vi "Main.vi"() -> ()   [LabVIEW 2020]
uses:
  Global_Variable/Global.vi
  Database/Global1.vi
  Global_Variable/A131258.vi
  <userlib>/_MGI/Menu Building/MenuTypes/MenuStrip/MGI_MenuStrip.lvclass
  <userlib>/_MGI/Menu Building/MenuItemStatusChange/MGI_MenuItemStatusChange.lvclass
  System.Windows.Forms
panel:
  in  "表格控件":string[][](table)
  out "上序状态":string
  in  "Andon":enum32{"未选择", "缺料报警", "质量报警", "故障报警"}(radio)
  in  "菜单":refnum<k24>(container)
  out "试验计时":u16
  out "工位传感器码":string
  out "生产数量":i32
  out "合格数量":i32
  out "userStatus":string caption="用户状态"
  out "userName":string caption="用户名"
  out "connectionMode":string caption="联机类型"
  out "产品型号":string
  in  "更换产品":refnum<vi>
  out "提示信息":string
  out "错误":bool
  out "时间字符串":string
  out "日期字符串":string
  out "自动":bool
  # "上转向轴组件压装"
  # "实验项目"
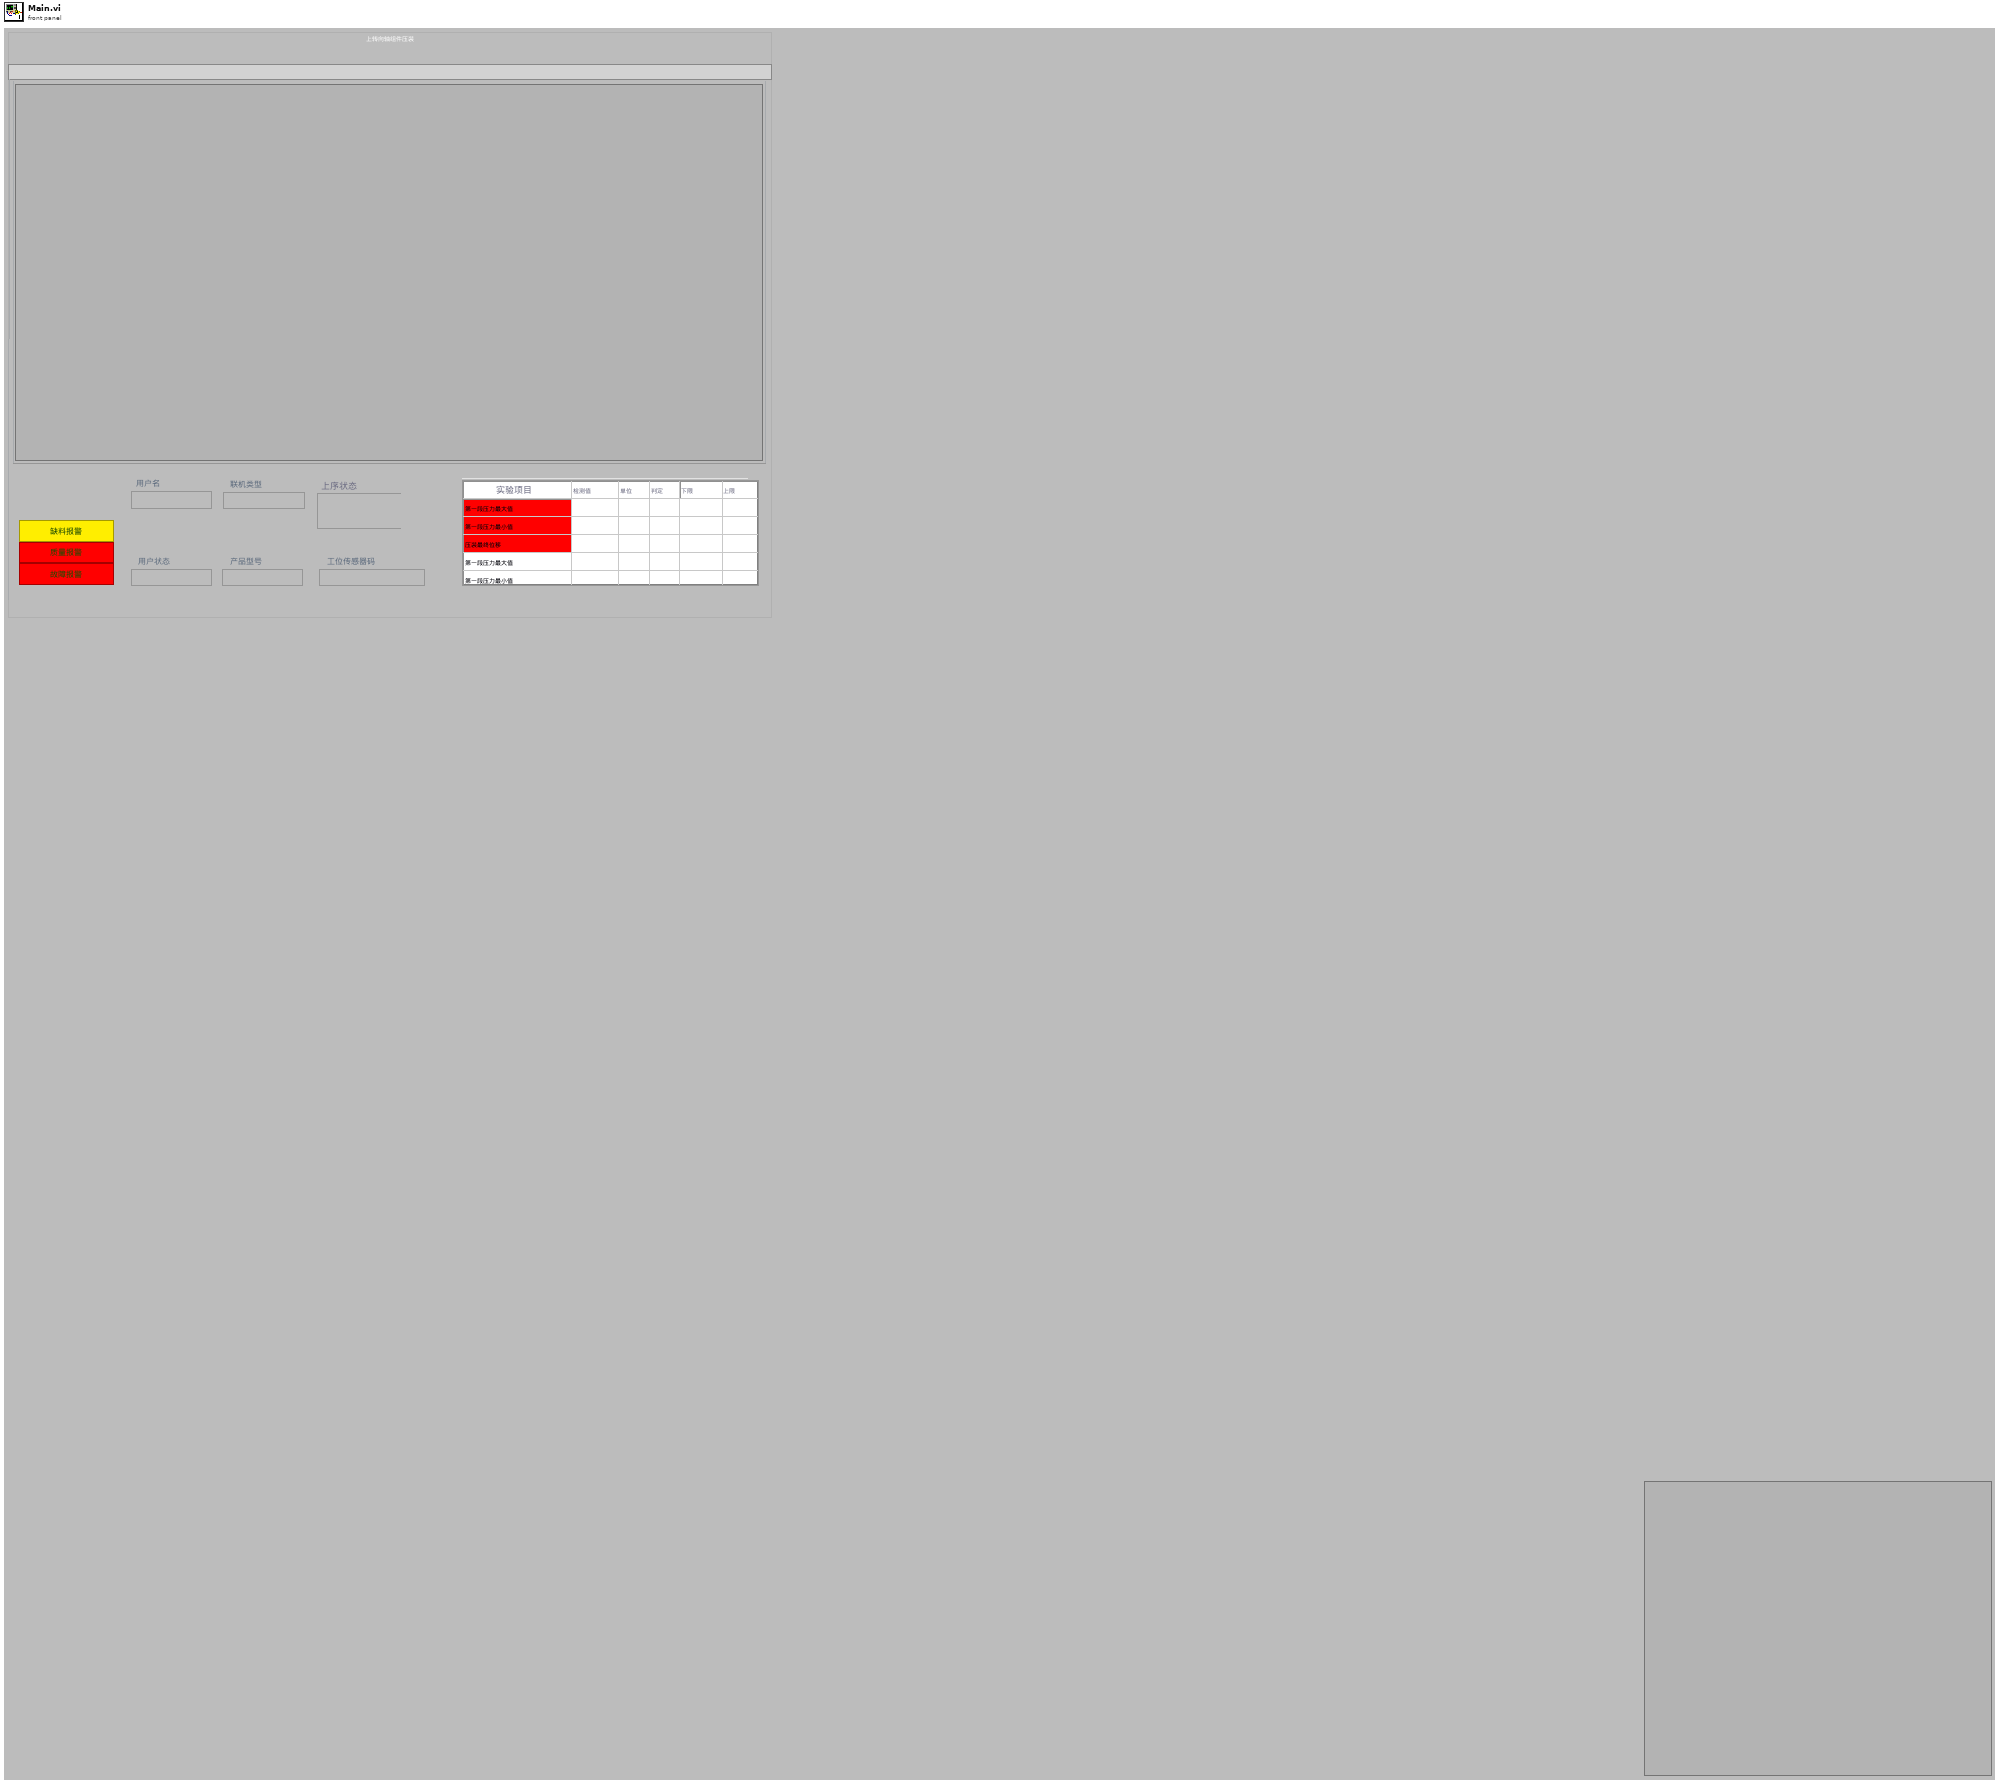
[diagram p1: front panel]
types:
  T1 = enum32{"Invalid", "Standard", "Closed", "Hidden", "Minimized", "Maximized"}
  T2 = cluster{"设备名称":string, "操作人员":string, "设备状态":enum16{"设备离线", "设备正常", "设备缺料", "设备故障", "质量报警"}, "附加信息":string}
  T3 = enum32{"invalid app kind", "Development System", "Run Time System", "Student Edition", "Embedded LabVIEW", "Evaluation", "Custom"}
  T4 = cluster{"用户编号":string, "用户名":string, "用户密码(密文)":string, "用户权限":string}
  T5 = cluster{"Core":cluster{"Current VI Reference":refnum<vi>, "Close Panel on Exit?":bool}, "Your Boolean data":bool, "Your string data":string}
  T6 = cluster{"Current VI Reference":refnum<vi>, "Close Panel on Exit?":bool}
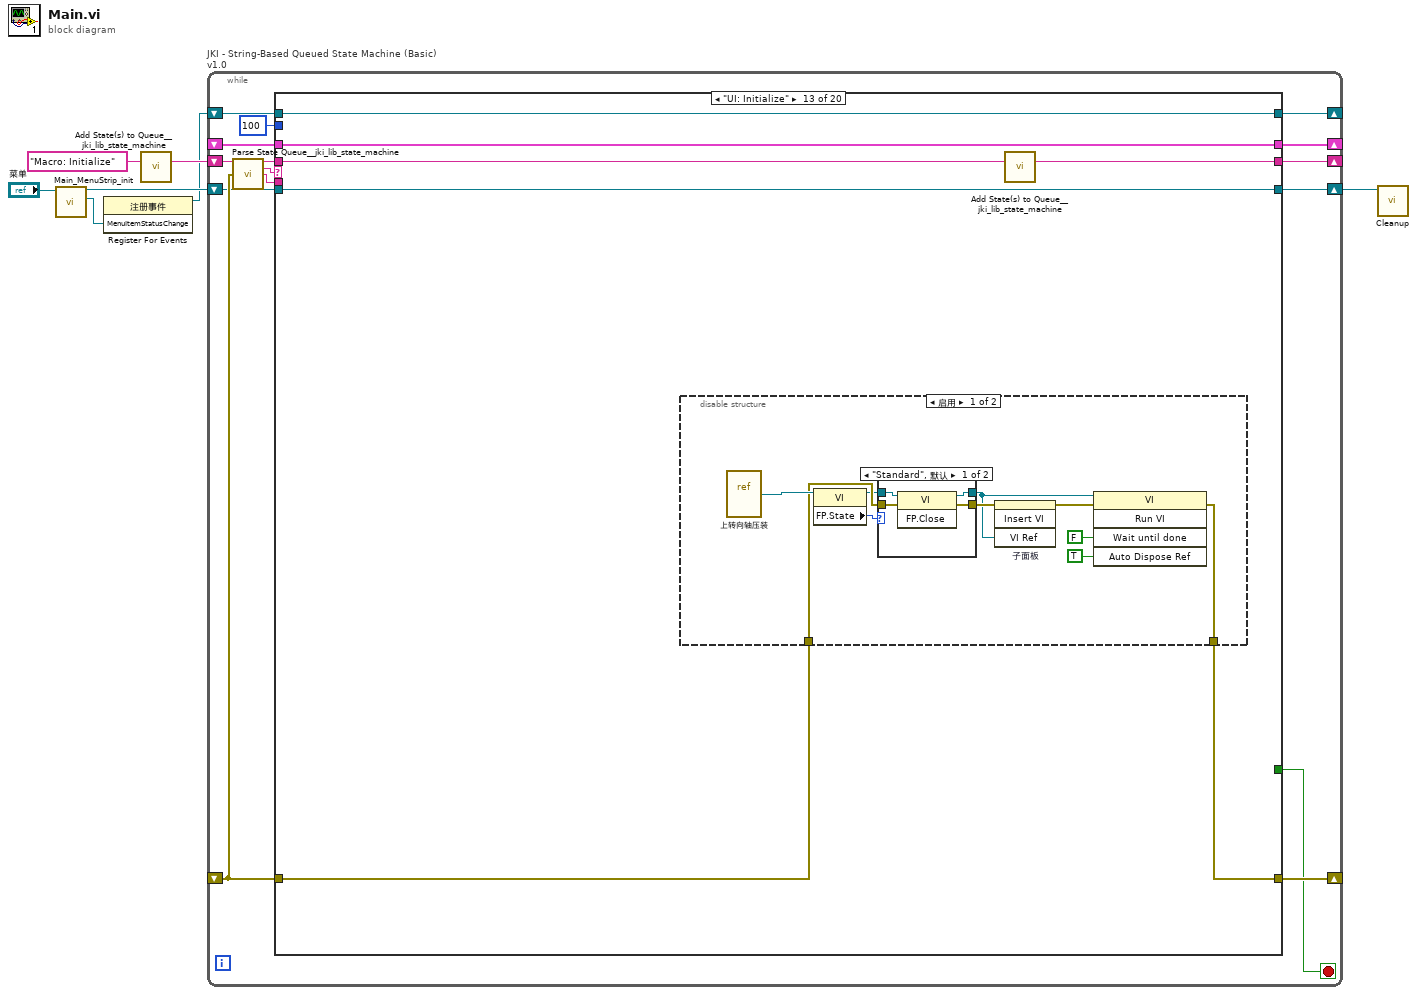
[diagram p0: block diagram]
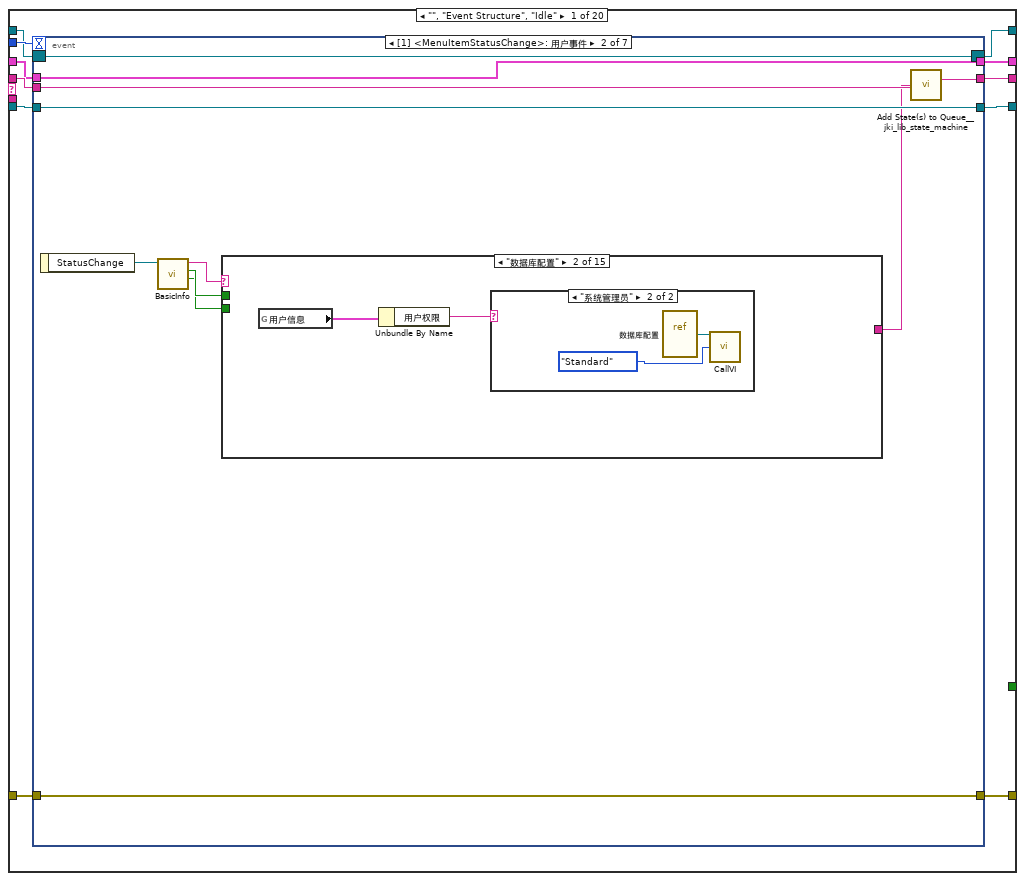
[diagram p2: hidden frame]
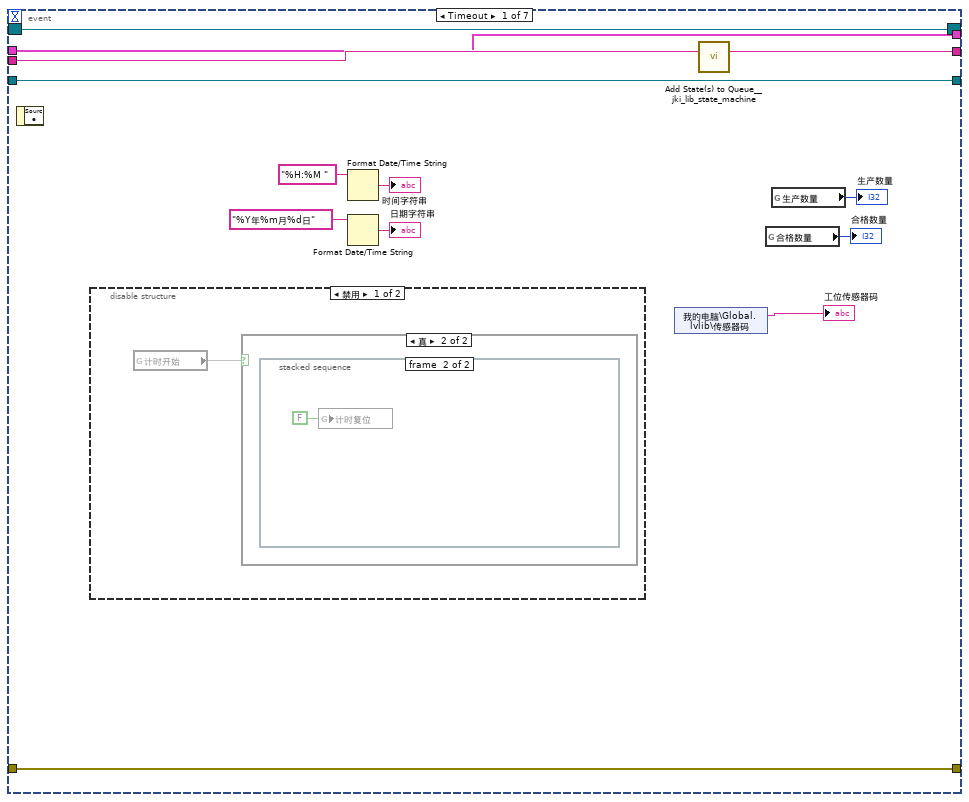
[diagram p3: hidden frame]
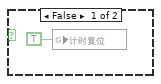
[diagram p4: hidden frame]
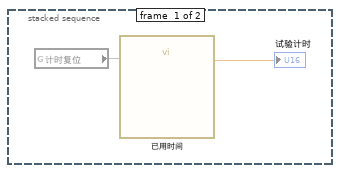
[diagram p5: hidden frame]
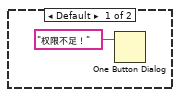
[diagram p8: hidden frame]
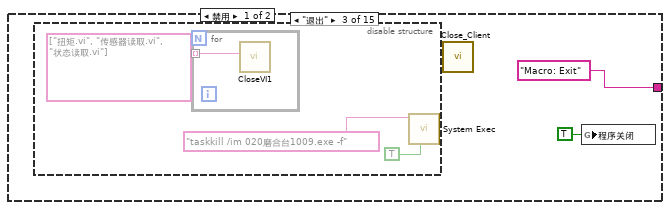
[diagram p9: hidden frame]
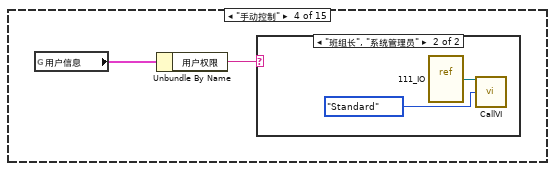
[diagram p11: hidden frame]
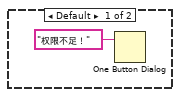
[diagram p12: hidden frame]
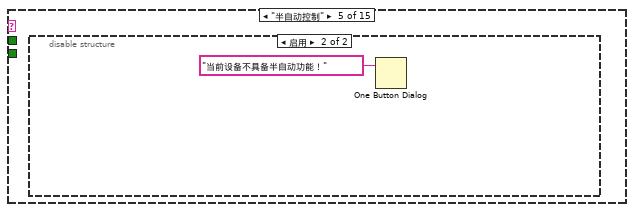
[diagram p13: hidden frame]
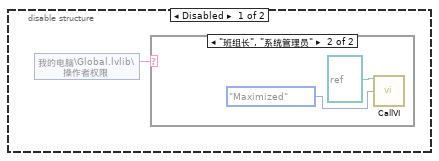
[diagram p14: hidden frame]
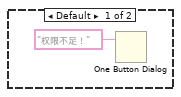
[diagram p15: hidden frame]
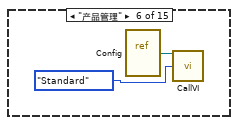
[diagram p16: hidden frame]
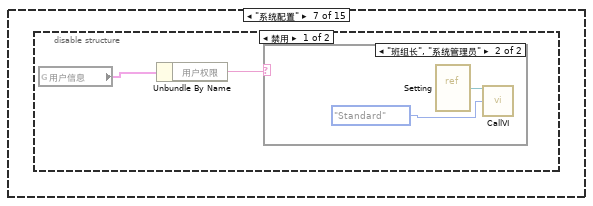
[diagram p17: hidden frame]
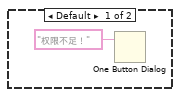
[diagram p18: hidden frame]
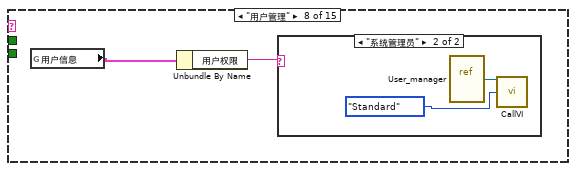
[diagram p20: hidden frame]
diagram:
  n1 = call "Main_MenuStrip_init.vi"("MenuStrip"="菜单") -> ("MenuItemStatusChange"=w2:refnum<user-event>, "Menu out"=w4:refnum<class "MGI_MenuStrip.lvclass">)  [unwired: 9 in]
  n2 = register-events(w2) -> (reference out=w1:refnum<event-registration>)  [unwired: 2 in, 1 out]
  n3 = call <vilib>:"Add State(s) to Queue__jki_lib_state_machine.vi"("State(s) in (\"\")"="Macro: Initialize") -> ("States Out"=w7:string)  [unwired: 14 in]
  n4 = while "JKI - String-Based Queued State Machine (Basic) v1.0" {
    shift-right: [w16] -> _
    shift-left: _ -> [w15]
    shift-right: [w18] -> _
    shift-left: _ -> [w13]
    shift-right: [w17] -> _
    shift-left: w7 -> [w19]
    shift-right: [w11] -> w3
    shift-left: w4 -> [w12]
    shift-right: [w9] -> _
    shift-left: w1 -> [w8]
    stop <- w10 stop-if-true
    n5 = call <vilib>:"Parse State Queue__jki_lib_state_machine.vi"("State Queue"=w19, "Error In (no error)"=w13) -> ("Remaining States"=w21:string, "Current State"=w22:string, "Arguments"=w20:string)  [unwired: 11 in]
    n6 = case shown="\"UI: Initialize\"" w22 {
      selector: w22 -> [_ _ w190 _ _ _ _ _ _ _ _ _ _ _ _ _ _ _ _ _]
      tunnel: w21 -> [w33 w187 w194 w214 w222 w229 w235 w238 w246 w257 w265 w271 w278 w302 w343 w351 w364 w392 w399 w411]
      tunnel: w20 -> [_ _ _ _ _ _ _ _ _ _ _ _ _ _ _ w346 w358 _ _ _]
      tunnel: w15 -> [w31 w184 w192 w205 w219 w227 w232 w239 w243 _ w260 w268 w276 w300 w340 w349 w360 w389 w396 w408]
      tunnel: [w30 w185 w196 w211 errorcluster {"status"=FALSE, "code"=0, "source"=""} ("error out") w226 w233 w236 w244 w254 w261 w269 w275 w298 w341 w347 w361 w390 w397 w409] -> w18
      tunnel: w13 -> [w29 w185 w195 w211 w218 w226 w233 w236 w244 w254 w262 w269 w272 w298 w341 w348 w362 w390 w397 w409]
      tunnel: [w32 w186 w193 w213 w221 w228 w234 w238 w245 w256 w264 w270 w277 w301 w342 w350 w363 w391 w398 w410] -> w17
      tunnel: [w28 w184 w192 w212 w219 w227 w232 w239 w243 w255 w260 w268 w276 w300 w340 w349 w360 w389 w396 w408] -> w16
      tunnel: 100 ("Timeout") -> [w27 _ _ _ _ _ _ _ _ _ _ _ _ _ _ _ _ _ _ _]
      tunnel: w12 -> [w26 w183 w189 w202 w216 w225 w231 w237 w242 w249 w259 w267 w274 w299 w339 w345 w357 w388 w394 w401]
      tunnel: [w25 w183 w189 w202 w216 w225 w231 w237 w242 w249 w259 w267 w274 w299 w339 w345 w357 w388 w394 w401] -> w11
      tunnel: [_ _ _ _ _ TRUE _ _ _ _ _ _ _ _ _ _ _ _ _ _] -> w10
      tunnel: [w23 w182 w188 w201 w215 w223 w230 w240 w241 w250 w258 w266 w273 w297 w336 w344 w356 w387 w393 w400] -> w9
      tunnel: w8 -> [w24 w182 w188 w201 w215 w223 w230 w240 w241 w250 w258 w266 w273 w297 w336 w344 w356 w387 w393 w400]
      frame "", "Event Structure", "Idle" {
        n7 = event shown="[1] <MenuItemStatusChange>: 用户事件" {
          selector: w24 -> [w36 w52 w127 w136 w144 w152 _]
          dyn-events: [w36 w52 w127 w136 w144 w152 _] -> w23
          timeout: w27 -> [_ _ _ _ _ _ _]
          tunnel: w33 -> [w46 w61 w124 w140 w150 w154 w176]
          tunnel: [w45 w59 w125 w141 w149 w155 w176] -> w32
          tunnel: w31 -> [w44 w60 w126 w142 w147 w157 w177]
          tunnel: [w37 w62 w122 w139 w148 w156 w174] -> w30
          tunnel: w29 -> [w37 w62 w122 w139 w148 w156 w174]
          tunnel: [w44 w60 w126 w142 w147 w157 w177] -> w28
          tunnel: w26 -> [w35 w55 w123 _ _ _ w175]
          tunnel: [w35 w55 w123 _ _ _ w175] -> w25
          event Timeout {
            n8 = event-data() -> ()  [unwired: 1 in, 1 out]
            n9 = disable-structure shown="禁用" {
              frame Disabled {
                n10 = global read "Global.vi" "计时开始"() -> (w47)
                n11 = case shown="真" w47 {
                  frame False {
                    n12 = global write "Global.vi" "计时复位"(TRUE ("计时复位")) -> ()
                  }
                  frame True {
                    n13 = stacked-sequence {
                      frame #0 {
                        n14 = global read "Global.vi" "计时复位"() -> (w49)
                        n15 = call "已用时间"("Reset"=w49) -> ("Elapsed Time (s)"=→"试验计时":dbl)  [unwired: 11 in, 7 out]
                      }
                      frame #1 {
                        n16 = global write "Global.vi" "计时复位"(FALSE ("计时复位")) -> ()
                      }
                    }
                  }
                }
              }
              frame Enabled {
              }
            }
            n17 = Format Date/Time String(time format string (%c)="%H:%M ") -> (date/time string=→"时间字符串":string)  [unwired: 2 in]
            n18 = Format Date/Time String(time format string (%c)="%Y年%m月%d日") -> (date/time string=→"日期字符串":string)  [unwired: 2 in]
            n19 = shared-variable "我的电脑\\Global.lvlib\\传感器码"() -> (→"工位传感器码":string)  [unwired: 1 in, 1 out]
            n20 = call <vilib>:"Add State(s) to Queue__jki_lib_state_machine.vi"("State(s) in (\"\")"=w46) -> ("States Out"=w45:string)  [unwired: 14 in]
            n21 = global read "Global.vi" "合格数量"() -> (→"合格数量":i32)
            n22 = global read "Global.vi" "生产数量"() -> (→"生产数量":i32)
          }
          event User Event {
            n23 = event-data() -> ("StatusChange"=w53:refnum<class "MGI_MenuItemStatusChange.lvclass">)  [unwired: 1 in]
            n24 = call <userlib>:"BasicInfo.vi"("MGI_MenuItemStatusChange in"=w53) -> ("Enabled?"=w56:bool, "Checked?"=w57:bool, "Tag"=w58:string)  [unwired: 7 in, 1 out]
            n25 = case shown="\"数据库配置\"" w58 {
              tunnel: w57 -> [_ _ _ _ _ _ _ _ _ _ _ _ _ _ _]
              tunnel: w56 -> [_ _ _ _ _ _ _ _ _ _ _ _ _ _ _]
              tunnel: [_ _ "Macro: Exit" _ _ _ _ _ _ _ _ _ _ _ _] -> w54
              frame "假", Default {
              }
              frame "数据库配置" {
                n26 = global read "Global1.vi" "用户信息"() -> (w63:T4)
                n27 = Unbundle By Name(w63) -> ("用户权限"=w64:string)
                n28 = case shown="\"系统管理员\"" w64 {
                  frame Default {
                    n29 = One Button Dialog(message="权限不足！" ("消息")) -> ()  [unwired: 1 in, 1 out]
                  }
                  frame "系统管理员" {
                    n30 = vi-ref "数据库配置.vi"() -> (w67:refnum<vi>)
                    n31 = call "CallVI.vi"("VI引用"=w67, "状态"=T1."Standard") -> ()  [unwired: 11 in, 3 out]
                  }
                }
              }
              frame "退出" {
                n32 = disable-structure shown="禁用" {
                  frame Disabled {
                    n33 = for {
                      tunnel: string[] ["扭矩.vi", "传感器读取.vi", "状态读取.vi"] -> [w73] mode=indexing
                      n34 = call "CloseVI1.vi"("名称或相对路径"=w73) -> ()  [unwired: 10 in, 1 out]
                    }
                    n35 = call <vilib>:"System Exec.vi"("run minimized? (F)"=TRUE, "command line"="taskkill /im 020磨合台1009.exe -f") -> ()  [unwired: 6 in, 4 out]
                  }
                  frame Enabled {
                  }
                }
                n36 = call "Close_Client.vi"() -> ()  [unwired: 12 in]
                n37 = global write "Global.vi" "程序关闭"(TRUE ("程序关闭")) -> ()
              }
              frame "手动控制" {
                n38 = global read "Global1.vi" "用户信息"() -> (w74:T4)
                n39 = Unbundle By Name(w74) -> ("用户权限"=w75:string)
                n40 = case shown="\"班组长\", \"系统管理员\"" w75 {
                  frame Default {
                    n41 = One Button Dialog(message="权限不足！" ("消息")) -> ()  [unwired: 1 in, 1 out]
                  }
                  frame "班组长", "系统管理员" {
                    n42 = vi-ref "111_IO.vi"() -> (w78:refnum<vi>)
                    n43 = call "CallVI.vi"("VI引用"=w78, "状态"=T1."Standard") -> ()  [unwired: 11 in, 3 out]
                  }
                }
              }
              frame "半自动控制" {
                n44 = disable-structure shown="启用" {
                  frame Disabled {
                    n45 = shared-variable "我的电脑\\Global.lvlib\\操作者权限"() -> (w79:string)  [unwired: 1 in, 1 out]
                    n46 = case shown="\"班组长\", \"系统管理员\"" w79 {
                      frame Default {
                        n47 = One Button Dialog(message="权限不足！" ("消息")) -> ()  [unwired: 1 in, 1 out]
                      }
                      frame "班组长", "系统管理员" {
                        n48 = call "CallVI.vi"("VI引用"=refnum<vi> refnum, "状态"=T1."Maximized") -> ()  [unwired: 11 in, 3 out]
                      }
                    }
                  }
                  frame Enabled {
                    n49 = One Button Dialog(message="当前设备不具备半自动功能！" ("消息")) -> ()  [unwired: 1 in, 1 out]
                  }
                }
              }
              frame "产品管理" {
                n50 = vi-ref "Config.vi"() -> (w85:refnum<vi>)
                n51 = call "CallVI.vi"("VI引用"=w85, "状态"=T1."Standard") -> ()  [unwired: 11 in, 3 out]
              }
              frame "系统配置" {
                n52 = disable-structure shown="禁用" {
                  frame Disabled {
                    n53 = global read "Global1.vi" "用户信息"() -> (w86:T4)
                    n54 = Unbundle By Name(w86) -> ("用户权限"=w87:string)
                    n55 = case shown="\"班组长\", \"系统管理员\"" w87 {
                      frame Default {
                        n56 = One Button Dialog(message="权限不足！" ("消息")) -> ()  [unwired: 1 in, 1 out]
                      }
                      frame "班组长", "系统管理员" {
                        n57 = vi-ref "Setting.vi"() -> (w90:refnum<vi>)
                        n58 = call "CallVI.vi"("VI引用"=w90, "状态"=T1."Standard") -> ()  [unwired: 11 in, 3 out]
                      }
                    }
                  }
                  frame Enabled {
                  }
                }
              }
              frame "用户管理" {
                n59 = global read "Global1.vi" "用户信息"() -> (w91:T4)
                n60 = Unbundle By Name(w91) -> ("用户权限"=w92:string)
                n61 = case shown="\"系统管理员\"" w92 {
                  frame Default {
                    n62 = One Button Dialog(message="权限不足！" ("消息")) -> ()  [unwired: 1 in, 1 out]
                  }
                  frame "系统管理员" {
                    n63 = vi-ref "User_manager.vi"() -> (w95:refnum<vi>)
                    n64 = call "CallVI.vi"("VI引用"=w95, "状态"=T1."Standard") -> ()  [unwired: 11 in, 3 out]
                  }
                }
              }
              frame "编码规则" {
                n65 = global read "Global1.vi" "用户信息"() -> (w96:T4)
                n66 = Unbundle By Name(w96) -> ("用户权限"=w97:string)
                n67 = case shown="\"班组长\", \"工艺管理员\", \"系统管理员\"" w97 {
                  frame Default {
                    n68 = One Button Dialog(message="权限不足！" ("消息")) -> ()  [unwired: 1 in, 1 out]
                  }
                  frame "班组长", "工艺管理员", "系统管理员" {
                    n69 = vi-ref "编码规则设置.vi"() -> (w100:refnum<vi>)
                    n70 = call "CallVI.vi"("VI引用"=w100, "状态"=T1."Standard") -> ()  [unwired: 11 in, 3 out]
                  }
                }
              }
              frame "易损件管理" {
                n71 = vi-ref "易损件管理.vi"() -> (w102:refnum<vi>)
                n72 = call "CallVI.vi"("VI引用"=w102, "状态"=T1."Standard") -> ()  [unwired: 11 in, 3 out]
              }
              frame "物料批次管理" {
                n73 = vi-ref "批次管理.vi"() -> (w104:refnum<vi>)
                n74 = call "CallVI.vi"("VI引用"=w104, "状态"=T1."Standard") -> ()  [unwired: 11 in, 3 out]
              }
              frame "报表" {
                n75 = call "文件对话框"("start path"=path "D:/report", "prompt"="打开报表", "pattern (all files)"="*.doc;*.docx", "pattern label"="Word 文档") -> ("selected path"=w105:path, "error out"=w106:errorcluster)  [unwired: 8 in, 2 out]
                n76 = case shown="无错误" w106 {
                  selector: w106 -> [w112 w114]
                  tunnel: w105 -> [w113 _]
                  frame No Error {
                    w111 = 1 items=["Normal", "Maximize", "Minimize"] ("cpubbs_WindowState")
                    n77 = call "Open_Word.vi"("File Path"=w113, "cpubbs_WindowState"=w111, "错误输入（无错误）"=w112) -> ()  [unwired: 12 in, 1 out]
                  }
                  frame Error {
                    n78 = call <vilib>:"Clear Errors.vi"("error in (no error)"=w114) -> ()  [unwired: 5 in, 2 out]
                  }
                }
              }
              frame "报警信息" {
                n79 = vi-ref "报警信息.vi"() -> (w116:refnum<vi>)
                n80 = call "CallVI.vi"("VI引用"=w116, "状态"=T1."Standard") -> ()  [unwired: 11 in, 3 out]
              }
              frame "关于" {
                n81 = vi-ref "About.vi"() -> (w118:refnum<vi>)
                n82 = call "CallVI.vi"("VI引用"=w118, "状态"=T1."Standard") -> ()  [unwired: 11 in, 3 out]
              }
              frame "操作演示" {
                n83 = call <vilib>:"Application Directory.vi"() -> ("Application Directory"=w121:path)
                n84 = Build Path(base path=w121, name or relative path="操作演示" ("名称或相对路径")) -> (appended path=w120:path)
                n85 = call "自动播放ppt.vi"("路径"=w120) -> ()  [unwired: 10 in, 1 out]
              }
            }
            n86 = call <vilib>:"Add State(s) to Queue__jki_lib_state_machine.vi"("State(s) in (\"\")"=w61, "State(s) at Back (\"\")"=w54) -> ("States Out"=w59:string)  [unwired: 13 in]
          }
          event "自动": Mouse Down {
            n87 = event-data() -> ()  [unwired: 1 in, 1 out]
            n88 = disable-structure shown="禁用" {
              frame Disabled {
                n89 = local read "自动"() -> (w128:bool)
                n90 = case shown="假" w128 {
                  frame False {
                    n91 = call "设备状态.vi"() -> ("Status_Read"=w129:i16)  [unwired: 11 in]
                    n92 = case shown="5" w129 {
                      frame 0, Default {
                        n93 = One Button Dialog(message="请复位！" ("消息")) -> ()  [unwired: 1 in, 1 out]
                      }
                      frame 5 {
                      }
                    }
                  }
                  frame True {
                    n94 = Two Button Dialog(message="确定要退出自动？" ("消息")) -> (T button?=w131:bool)  [unwired: 2 in]
                    n95 = case shown="真" w131 {
                      frame False {
                      }
                      frame True {
                        n96 = vi-ref "Auto.vi"() -> (w135:refnum<vi>)
                        n97 = invoke class="VI" method="Ctrl Val.Set"(reference=w135, "Control Name"="STEP" ("控件名"), "Value"="退出自动" ("控件名")) -> ()  [unwired: 2 in, 5 out]
                      }
                    }
                  }
                }
              }
              frame Enabled {
              }
            }
            n98 = call <vilib>:"Add State(s) to Queue__jki_lib_state_machine.vi"("State(s) in (\"\")"=w124) -> ("States Out"=w125:string)  [unwired: 14 in]
          }
          event "错误": Mouse Down {
            n99 = event-data() -> ()  [unwired: 1 in, 8 out]
            n100 = vi-ref "报警信息.vi"() -> (w138:refnum<vi>)
            n101 = call "CallVI.vi"("VI引用"=w138, "状态"=T1."Standard") -> ()  [unwired: 11 in, 3 out]
            n102 = call <vilib>:"Add State(s) to Queue__jki_lib_state_machine.vi"("State(s) in (\"\")"=w140) -> ("States Out"=w141:string)  [unwired: 14 in]
          }
          event Panel Close? {
            w143 = TRUE ("程序关闭")
            n103 = event-data() -> ()  [unwired: 1 in, 1 out]
            n104 = global write "Global.vi" "程序关闭"(w143) -> ()
            n105 = call <vilib>:"Add State(s) to Queue__jki_lib_state_machine.vi"("State(s) in Front (\"\")"="S7: Stop\nMacro: Exit", "State(s) in (\"\")"=w150) -> ("States Out"=w149:string)  [unwired: 13 in]
            n106 = Quit LabVIEW(quit? (T)=w143) -> ()
            n107 = event-data("Discard?"=TRUE) -> ()  [unwired: 1 in, 1 out]
          }
          event "更换产品": Value Change {
            n108 = event-data() -> ("NewVal"=w153:refnum<vi>)  [unwired: 1 in, 5 out]
            n109 = stacked-sequence {
              tunnel: w153 -> [w166]
              tunnel: ["Idle"] -> w151
              frame #0 {
                n110 = disable-structure shown="禁用" {
                  disable-tunnel: w166 -> [w168 _]
                  frame Disabled {
                    n111 = control-ref of="子面板"() -> (w167:refnum<vi>)
                    n112 = call "Call_SubPanal.vi"("VI引用句柄"=w168, "SubPnl引用句柄"=w167) -> ()  [unwired: 9 in, 1 out]
                  }
                  frame Enabled {
                  }
                }
                n113 = vi-ref "上转向轴压装.vi"() -> (w163:refnum<vi>)
                n114 = invoke class="VI" method="Ctrl Val.Get"(reference=w163, "Control Name"="标尺_Event" ("控件名")) -> ("Get Control Value Variant"=w162:variant)  [unwired: 2 in, 3 out]
                n115 = shared-variable "我的电脑\\Global.lvlib\\产品型号"() -> (w158:string)  [unwired: 1 in, 1 out]
                n116 = Variant To Data(type=refnum<user-event> refnum ("标尺_Event"), Variant=w162) -> (data=w159:refnum<user-event>, error out=w160:errorcluster)  [unwired: 1 in]
                n117 = Generate User Event(user event=w159, event data cluster=w158, error in=w160) -> ()  [unwired: 1 in, 2 out]
                n118 = local write "产品型号"(w158) -> ()
              }
            }
            n119 = call <vilib>:"Add State(s) to Queue__jki_lib_state_machine.vi"("State(s) in Front (\"\")"=w151, "State(s) in (\"\")"=w154) -> ("States Out"=w155:string)  [unwired: 13 in]
          }
          event "Andon": Value Change {
            n120 = event-data() -> ("NewVal"=w173:enum32{"未选择", "缺料报警", "质量报警", "故障报警"})  [unwired: 1 in]
            n121 = case shown="\"故障报警\"" w173 {
              tunnel: [enum16{"设备离线", "设备正常", "设备缺料", "设备故障", "质量报警"}."设备正常" ("设备状态") enum16{"设备离线", "设备正常", "设备缺料", "设备故障", "质量报警"}."设备缺料" ("设备状态") enum16{"设备离线", "设备正常", "设备缺料", "设备故障", "质量报警"}."质量报警" ("设备状态") enum16{"设备离线", "设备正常", "设备缺料", "设备故障", "质量报警"}."设备故障" ("设备状态")] -> w171
              frame "未选择", Default {
              }
              frame "缺料报警" {
              }
              frame "质量报警" {
              }
              frame "故障报警" {
              }
            }
            n122 = local read "userName"() -> (w170:string)
            n123 = Bundle By Name(cluster=T2 {"设备名称"="上转向轴组件装配", "操作人员"="", "设备状态"=enum."设备离线", "附加信息"=""} ("设备信息"), "操作人员"=w170, "设备状态"=w171) -> (w169:T2)
            n124 = call "Change_Client.vi"("设备信息"=w169) -> ()  [unwired: 10 in, 1 out]
          }
        }
      }
      frame "---------- Core ----------" {
        n125 = call <vilib>:"Add State(s) to Queue__jki_lib_state_machine.vi"("State(s) in (\"\")"=w187) -> ("States Out"=w186:string)  [unwired: 14 in]
      }
      frame Default {
        w199 = 42 items=["No error", "Argument error", "Memory is full", "Out of zone", "End of file", "File already open", "Generic file I/O error", "File not found", "File permission error", "Disk is full", "Duplicate path", "Too many files open", "System feature not enabled", "Resource file not found", "Cannot add resource", "Resource not found", "Image not found", "Image memory error", "Pen does not exist", "Config type invalid", "Config token not found", "Config parse error", "Config memory error", "Bad external code format", "Bad external code offset", "External code not present", "Null window", "Destroy window error", "Null menu", "Print aborted", "Bad print record", "Print driver error", "Windows error during printing", "Memory error during printing", "Print dialog error", "Generic print error", "Invalid device refnum", "Device not found", "Device parameter error", "Device unit error", "Cannot open device", "Device call aborted", "Generic error", "Cancelled by user", "Object ID too low", "Object ID too high", "Object not in heap", "Unknown heap", "Unknown object (invalid DefProc)", "Unknown object (DefProc not in table)", "Message out of range", "Invalid (null) method", "Unknown message", "Manager call not supported", "Bad address", "Network operation in progress", "Network operation timed out", "Connection is busy", "Network attribute not supported", "Network error", "Address in use", "System out of memory", "Connection aborted", "Connection refused", "Not connected", "Already connected", "Connection closed", "Initialization error (interapplication manager)", "Bad occurrence", "Wait on unbound occurrence handler", "Occurrence queue overflow", "Datalog type conflict", "Unused", "Unrecognized type (interapplication manager)", "Memory corrupt", "Failed to make temporary DLL", "Old CIN version", "Drag socket not found", "Failed to load drop-object", "Failed to register OLE object", "Failed to release OLE object", "Format specifier type mismatch", "Unknown format specifier", "Too few format specifiers", "Too many format specifiers", "Scan failed", "Newer CIN version", "Error converting to variant", "Runtime menu error", "Password tampered", "Variant attribute not found", "Incompatible variant data type", "Event data is not available", "Event Store is not present", "Occurrence is not found", "Event Queue is not created", "Event info is not available", "Refnum passed is NULL", "Error retrieving Class GUID", "Error retrieving CoClass GUID", "Error retrieving TypeLib GUID.", "Bad built application magic bytes.", "Specific driver is different from the specific driver associated with the Logical Name.", "There is no session opened to the class driver.", "Max Error", "MAX - Error with config objects", "MAX - Error loading configuration", "MAX - Group not supported"]
        # "Current State"
        n126 = Format Into String(format string="Software Exception: Unhandled State \"%s\"." ("message"), error in=w195, w190) -> (resulting string=w198:string, error out=w197:errorcluster)  [unwired: 1 in]
        n127 = call <vilib>:"Error Cluster From Error Code.vi"("show call chain? (False)"=TRUE, "error in (no error)"=w197, "error message (\"\")"=w198, "error code (0)"=w199) -> ("error out"=w196:errorcluster)  [unwired: 5 in]
        n128 = call <vilib>:"Add State(s) to Queue__jki_lib_state_machine.vi"("State(s) in (\"\")"=w194) -> ("States Out"=w193:string)  [unwired: 14 in]
      }
      frame "Initialize Core Data" {
        # "originally closed?"
        # "exe?"
        n129 = property class="VI"() -> ("Front Panel.Open"=w210:bool)  [unwired: 2 in, 2 out]
        n130 = property class="App"() -> ("App.Kind"=w209:T3)  [unwired: 2 in, 2 out]
        n131 = control-ref of="Current VI Reference"() -> (w203:refnum<vi>)
        n132 = Not(x=w210) -> (.not. x?=w207:bool)
        n133 = Equal?(x=w209, y=T3."Run Time System" ("Application:Kind")) -> (x = y?=w206:bool)
        n134 = Or(x=w207, y=w206) -> (x .or. y?=w204:bool)
        n135 = Bundle By Name(cluster=w205, "Core.Current VI Reference"=w203, "Core.Close Panel on Exit?"=w204) -> (w212:T5)
        n136 = call <vilib>:"Add State(s) to Queue__jki_lib_state_machine.vi"("State(s) in (\"\")"=w214) -> ("States Out"=w213:string)  [unwired: 14 in]
      }
      frame "Error Handler" {
        n137 = call <vilib>:"General Error Handler.vi"("error in (no error)"=w218) -> ()  [unwired: 10 in, 5 out]
        n138 = call <vilib>:"Add State(s) to Queue__jki_lib_state_machine.vi"("State(s) in Front (\"\")"="/* Post Error States", "State(s) in (\"\")"=w222) -> ("States Out"=w221:string)  [unwired: 13 in]
      }
      frame "Exit" {
        n139 = call <vilib>:"Add State(s) to Queue__jki_lib_state_machine.vi"("State(s) in (\"\")"=w229) -> ("States Out"=w228:string)  [unwired: 14 in]
        n140 = Quit LabVIEW() -> ()  [unwired: 1 in]
      }
      frame "--------- Library --------" {
        n141 = call <vilib>:"Add State(s) to Queue__jki_lib_state_machine.vi"("State(s) in (\"\")"=w235) -> ("States Out"=w234:string)  [unwired: 14 in]
      }
      frame "S7: Initialize" {
      }
      frame "---------- Data ----------" {
        n142 = call <vilib>:"Add State(s) to Queue__jki_lib_state_machine.vi"("State(s) in (\"\")"=w246) -> ("States Out"=w245:string)  [unwired: 14 in]
      }
      frame "Data: Initialize" {
        (unwired) FALSE ("计时结束")
        w251 = T6 {"Current VI Reference"=refnum, "Close Panel on Exit?"=FALSE}  # Core
        w253 = TRUE  # Your Boolean data
        w252 = ""  # Your string data
        n143 = call "Fit VI window to Largest Dec.vi"("border spacing (2 px)"=0) -> ()  [unwired: 5 in, 2 out]
        n144 = global write "Global.vi" "程序关闭"(FALSE ("程序关闭")) -> ()
        n145 = Bundle("Core"=w251, "Your Boolean data"=w253, "Your string data"=w252) -> (w255:T5)  [unwired: 1 in]
        n146 = call <vilib>:"Add State(s) to Queue__jki_lib_state_machine.vi"("State(s) in (\"\")"=w257) -> ("States Out"=w256:string)  [unwired: 14 in]
      }
      frame "Data: Cleanup" {
        n147 = Unbundle By Name(w260) -> ("Core.Current VI Reference"=w263:refnum<vi>)
        n148 = Close Reference(reference=w263, error in (no error)=w262) -> (error out=w261:errorcluster)
        n149 = call <vilib>:"Add State(s) to Queue__jki_lib_state_machine.vi"("State(s) in (\"\")"=w265) -> ("States Out"=w264:string)  [unwired: 14 in]
      }
      frame "---------- UI ----------" {
        # "Do not put any code in this frame.\n(It is a separator no-op. You can make a copy of this frame to create a new UI frame)"
        n150 = call <vilib>:"Add State(s) to Queue__jki_lib_state_machine.vi"("State(s) in (\"\")"=w271) -> ("States Out"=w270:string)  [unwired: 14 in]
      }
      frame "UI: Initialize" {
        n151 = disable-structure shown="启用" {
          disable-tunnel: [w285 _] -> w275
          disable-tunnel: w272 -> [w283 _]
          frame Enabled {
            n152 = vi-ref "上转向轴压装.vi"() -> (w284:refnum<vi>)
            n153 = property class="VI"(reference=w284) -> (reference out=w282:refnum<vi>, "FP.State"=w281:T1)  [unwired: 1 in, 1 out]
            n154 = case shown="\"Standard\", 默认" w281 {
              tunnel: w283 -> [w291 w293]
              tunnel: w282 -> [w292 w294]
              tunnel: [w290 w294] -> w279
              tunnel: [w289 w293] -> w280
              frame "Standard", Default {
                n155 = invoke class="VI" method="FP.Close"(reference=w292, error in=w291) -> (reference out=w290:refnum<vi>, error out=w289:errorcluster)  [unwired: 1 in, 1 out]
              }
              frame "Invalid", "Closed" {
              }
            }
            n156 = invoke on="子面板" class="SubPnl" method="Insert VI"(error in=w280, "VI Ref"=w279) -> (error out=w288:errorcluster)  [unwired: 2 in, 3 out]
            n157 = invoke class="VI" method="Run VI"(reference=w279, error in=w288, "Wait until done"=FALSE ("结束前等待"), "Auto Dispose Ref"=TRUE ("自动销毁引用")) -> (error out=w285:errorcluster)  [unwired: 1 in, 4 out]
          }
          frame Disabled {
            n158 = vi-ref "Auto.vi"() -> (w296:refnum<vi>)
            n159 = call "CallVI.vi"("VI引用"=w296, "状态"=T1."Maximized") -> ()  [unwired: 11 in, 3 out]
          }
        }
        n160 = call <vilib>:"Add State(s) to Queue__jki_lib_state_machine.vi"("State(s) in (\"\")"=w278) -> ("States Out"=w277:string)  [unwired: 14 in]
      }
      frame "UI: Init" {
        n161 = stacked-sequence {
          tunnel: w298 -> [_ _ _ _]
          frame #0 {
            w305 = -2
            n162 = control-ref of="表格控件"() -> (w310:refnum<vi>)
            n163 = global write "Global.vi" "程序关闭"(FALSE ("程序关闭")) -> ()
            n164 = for {
              N: 4 -> [_]
              tunnel: [cluster{"X":dbl[], "Y":dbl[]} {"X"=[], "Y"=[]}] -> w306 mode=indexing
            }
            n165 = Bundle(w305, w305) -> (w304:cluster{i32, i32})  [unwired: 1 in]
            n166 = property class="Tbl (严格)"(reference=w310, "Row Headers[]"=string[] [] ("行首字符串[]"), "Value"=string[][] [] ("值"), "Active Cell"=w304, "Cell BG Color"=u32 16777216 ("活动单元格:单元格背景色")) -> ()  [unwired: 1 in, 2 out]
            n167 = global read "A131258.vi" "上转向轴压装曲线"() -> (w311:refnum<vi>)
            n168 = property class="XYGraph"(reference=w311, "Value"=w306) -> ()  [unwired: 1 in, 2 out]
          }
          frame #1 {
            w320 = 0
            n169 = shared-variable "我的电脑\\Global.lvlib\\总成追溯码"("   " ("工位追溯码")) -> ()  [unwired: 1 in, 1 out]
            n170 = global write "Global.vi" "生产数量"(w320) -> ()
            n171 = global write "Global.vi" "合格数量"(w320) -> ()
            n172 = global read "Global1.vi" "用户信息"() -> (w315:T4)
            n173 = global read "Global1.vi" "联机模式"() -> (w314:enum16{"单机", "追溯"})
            n174 = Unbundle By Name(w315) -> ("用户名"=→"userName":string, "用户权限"=→"userStatus":string)
            n175 = case shown="\"追溯\"" w314 {
              tunnel: ["联网" ("connectionMode") "单机" ("connectionMode")] -> w321
              frame "追溯" {
              }
              frame "单机", Default {
              }
            }
            "connectionMode" <- w321
            "产品型号" <- "" ("产品型号")
          }
          frame #2 {
            n176 = control-ref of="表格控件"() -> (w325:refnum<vi>)
            n177 = control-ref of="提示信息"() -> (w327:refnum<vi>)
            n178 = control-ref of="自动"() -> (w328:refnum<vi>)
            n179 = control-ref of="错误"() -> (w329:refnum<vi>)
            n180 = control-ref of="更换产品"() -> (w326:refnum<vi>)
            n181 = global write "Global.vi" "提示信息"(w327) -> ()
            n182 = global write "Global.vi" "程序自动"(w328) -> ()
            n183 = global write "Global.vi" "报警图标"(w329) -> ()
            n184 = global write "Global.vi" "Result"(w325) -> ()
            n185 = global write "Global.vi" "更换产品"(w326) -> ()
            n186 = control-ref of="上序状态"() -> (w324:refnum<vi>)
            n187 = global write "Global.vi" "上序状态"(w324) -> ()
          }
          frame #3 {
            w330 = -2
            n188 = global read "Global.vi" "Result"() -> (w333:refnum<vi>)
            n189 = property class="Tbl"(reference=w333, "Row Headers[]"=string[] [], "Value"=string[][] []) -> ()  [unwired: 1 in, 2 out]
            n190 = Bundle(w330, w330) -> (w331:cluster{i32, i32})  [unwired: 1 in]
            n191 = call "Start_Client.vi"() -> ()  [unwired: 12 in]
            n192 = property class="Tbl"(reference=w333, "Active Cell"=w331, "Cell BG Color"=u32 16777216 ("活动单元格:单元格背景色")) -> ()  [unwired: 1 in, 2 out]
          }
        }
        n193 = call <vilib>:"Add State(s) to Queue__jki_lib_state_machine.vi"("State(s) in (\"\")"=w302) -> ("States Out"=w301:string)  [unwired: 14 in]
      }
      frame "UI: Config" {
        n194 = vi-ref "Config.vi"() -> (w338:refnum<vi>)
        n195 = call "CallVI.vi"("VI引用"=w338, "状态"=T1."Standard") -> ()  [unwired: 11 in, 3 out]
        n196 = call <vilib>:"Add State(s) to Queue__jki_lib_state_machine.vi"("State(s) in (\"\")"=w343) -> ("States Out"=w342:string)  [unwired: 14 in]
      }
      frame "UI: Cursor Set" {
        # "Argument"
        n197 = case shown="\"Idle\", 默认" w346 {
          tunnel: w348 -> [w353 w355]
          tunnel: [w352 w354] -> w347
          frame "Idle", Default {
            n198 = call <vilib>:"Unset Busy.vi"("error in (no error)"=w353) -> ("error out"=w352:errorcluster)  [unwired: 10 in]
          }
          frame "Busy" {
            n199 = call <vilib>:"Set Busy.vi"("error in (no error)"=w355) -> ("error out"=w354:errorcluster)  [unwired: 9 in, 1 out]
          }
        }
        n200 = call <vilib>:"Add State(s) to Queue__jki_lib_state_machine.vi"("State(s) in (\"\")"=w351) -> ("States Out"=w350:string)  [unwired: 14 in]
      }
      frame "UI: Front Panel State" {
        # "Argument"
        n201 = Unbundle By Name(w360) -> ("Core.Current VI Reference"=w359:refnum<vi>)
        n202 = case shown="\"Close\"" w358 {
          tunnel: w362 -> [w368 w381]
          tunnel: [w370 w382] -> w361
          tunnel: w359 -> [w369 w379]
          frame "Open", Default {
            n203 = property class="VI"(reference=w369, error in=w368) -> (reference out=w366:refnum<vi>, error out=w367:errorcluster, "Front Panel.Open"=w365:bool)
            n204 = case shown="假" w365 {
              tunnel: [w373 w376] -> w370
              tunnel: w367 -> [w372 w376]
              tunnel: w366 -> [w371 _]
              frame False {
                n205 = invoke class="VI" method="FP.Open"(reference=w371, error in=w372, "Activate"=TRUE, "State"=T1."Standard") -> (error out=w373:errorcluster)  [unwired: 1 in, 4 out]
              }
              frame True {
              }
            }
          }
          frame "Close" {
            n206 = property class="VI"(reference=w379, error in=w381) -> (reference out=w378:refnum<vi>, error out=w380:errorcluster, "Front Panel.Open"=w377:bool)
            n207 = case shown="真" w377 {
              tunnel: [w383 w386] -> w382
              tunnel: w380 -> [w383 w385]
              tunnel: w378 -> [_ w384]
              frame False {
              }
              frame True {
                n208 = invoke class="VI" method="FP.Close"(reference=w384, error in=w385) -> (error out=w386:errorcluster)  [unwired: 1 in, 2 out]
              }
            }
          }
        }
        n209 = call <vilib>:"Add State(s) to Queue__jki_lib_state_machine.vi"("State(s) in (\"\")"=w364) -> ("States Out"=w363:string)  [unwired: 14 in]
      }
      frame "---------- Macro ----------" {
        n210 = call <vilib>:"Add State(s) to Queue__jki_lib_state_machine.vi"("State(s) in (\"\")"=w392) -> ("States Out"=w391:string)  [unwired: 14 in]
      }
      frame "Macro: Initialize" {
        n211 = call <vilib>:"Add State(s) to Queue__jki_lib_state_machine.vi"("State(s) in Front (\"\")"="Data: Initialize\nInitialize Core Data\nS7: Initialize\nIdle\nUI: Init\nUI: Front Panel State >> Open\nUI: Initialize\nUI: Config", "State(s) in (\"\")"=w399) -> ("States Out"=w398:string)  [unwired: 13 in]
      }
      frame "Macro: Exit" {
        n212 = Unbundle By Name(w408) -> ("Core.Close Panel on Exit?"=w407:bool)
        n213 = Select(t="UI: Front Panel State >> Close", s=w407, f="") -> (s? t:f=w404:string)
        n214 = call <vilib>:"Add State(s) to Queue__jki_lib_state_machine.vi"("State(s) in (\"\")"=w404, "State(s) at Back (\"\")"="Data: Cleanup\nExit") -> ("States Out"=w402:string)  [unwired: 13 in]
        n215 = call <vilib>:"Add State(s) to Queue__jki_lib_state_machine.vi"("State(s) in Front (\"\")"=w402, "State(s) in (\"\")"=w411) -> ("States Out"=w410:string)  [unwired: 13 in]
      }
    }
  }
  n216 = call-dynamic "Cleanup.vi"("MenuStrip in"=w3) -> ()  [unwired: 10 in, 1 out]
